vi "UHR-Fleezers Control (host) - 10.5.vi"() -> ()   [LabVIEW 2010]
uses:
  <vilib>/Utility/miscctls.llb/LVPoint32TypeDef.ctl
  <vilib>/Utility/miscctls.llb/LVMinMaxIncTypeDef.ctl
  openfpgaref.8.6.ctl
  <vilib>/userDefined/High Color/nirio_resource_hc.ctl
  <vilib>/Platform/TimedLoop/XDataNode/XDataNode.xnode
  <vilib>/Platform/TimedLoop/XDataNode/timing_clust.ctl
  <vilib>/Platform/TimedLoop/XDataNode/nitl_modes.ctl
  <vilib>/Platform/TimedLoop/XDataNode/wakeup.ctl
  <vilib>/rvi/interface/nirviOpenFPGA/nirviOpenFPGA.xnode
  FPGA Bitfiles/UHR-FleezersInst_FPGATarget_UHR-FleezersCont_0F5B06C4.lvbitx
  UHR-Fleezers Control (fpga) - 10.3.vi
  <vilib>/rvi/ClientSDK/nirviWhatTheDeviceIsDoing.ctl
  <vilib>/rvi/interface/nirviMethod/nirviMethod.xnode
  <vilib>/rvi/interface/nirviReadWriteControl/nirviReadWriteControl.xnode
  <vilib>/rvi/interface/common/niFpgaNodeNameForErrorReporting.ctl
  <vilib>/rvi/errors/niLvFpgaWhatHappensToTopLevelVI.ctl
  <vilib>/express/express analysis/Spectral/XNode/ExpressSpectralMeasurementsBlockNode.xnode
  <vilib>/rvi/interface/nirviCloseFPGA/nirviCloseFPGA.xnode
  <vilib>/Instr/_visa.llb/VISA Configure Serial Port (Instr).vi
  <vilib>/FPGAPlugInAG/PCIe-7852R/niLvFpga_Open_PCIe-7852R.vi
  <vilib>/FPGAPlugInAG/PCIe-7852R/niLvFpga_Reset_PCIe-7852R.vi
  <vilib>/Utility/error.llb/Error Cluster From Error Code.vi
  <vilib>/rvi/errors/niLvFpgaAdjustHostInterfaceError.vi
  <vilib>/express/express analysis/Spectral/Block/exnSpectralBlock spectral measurements PSD poly.vi
  <vilib>/express/express analysis/Spectral/Block/exnSpectralBlock spectral measurements PSD WFM.vi
  <vilib>/Waveform/WDTOps.llb/WDT Append Waveforms DBL.vi
  <vilib>/FPGAPlugInAG/PCIe-7852R/niLvFpga_Abort_PCIe-7852R.vi
  <vilib>/FPGAPlugInAG/PCIe-7852R/niLvFpga_Close_PCIe-7852R.vi
  <vilib>/Analysis/NI_AALBase.lvlib
  <vilib>/Platform/TimedLoop/XDataNode/XDNodeRunTimeDep.lvlib
  <vilib>/vision/NI_Vision_Development_Module.lvlib
  NiFpgaLv.dll
  <vilib>/Utility/inputDevices.llb/mouseAcquire.vi
  User32.dll
  <vilib>/Utility/inputDevices.llb/closeMouse.vi
panel:
  out "Array":cluster{i32, i32, i32, i32}[](array[cluster])
  in  "radius":i32
  in  "clear markers":bool
  in  "trap\nmarkers?":bool
  out "x-y":u32=299
  in  "Sample Channel Flow":bool
  in  "Pump 3 contents":string="Left: ADig beads" caption="contents"
  in  "Pump 1 contents":string="Right: DNA beads" caption="contents"
  in  "Scripts":T1(tab)
  in  "Take Stepping Data":bool
  in  "Cap 1 Samp Flow ON":bool=TRUE
  in  "Cap 2 Samp Flow ON":bool=TRUE
  in  "Got DNA bead":bool
  in  "Got ADig bead":bool
  in  "Cap 2 Flow ON":bool=TRUE
  in  "Cap 1 Flow ON":bool=TRUE
  in  "Cap 2 T ON":bool=TRUE
  in  "Move Cap. 2 (ADig Left)":bool
  in  "Move Cap. 1 (DNA Right)":bool
  in  "Cal/Data Acq. Spot":bool
  in  "Dump Beads":bool
  in  "Lower Ch. Cap.":bool
  in  "Cap 1 T ON":bool=TRUE
  in  "Offset 2 Set":dbl=2.0
  in  "Offset 1 Set":dbl
  in  "Cal @ (MHz)":dbl=15.0
  in  "W/ Offset 1":bool=TRUE
  in  "Offset 1 Start (MHz)":dbl=13.0
  in  "W/ Offset 2":bool=TRUE
  in  "Offset 2 Start (MHz)":dbl=16.0
  in  "Move to Delta 2 (MHz)":dbl=13.0
  in  "Attempt Limit":dbl=30.0 caption="Limit"
  out "Attempts":dbl=1.0
  in  "Wait Before Save (s)":u32=1
  in  "Fish for Tether":bool
  in  "Closest Delta (MHz)":dbl=9.5 step=0.25
  in  "Stop F (pN)":dbl=3.0
  in  "Then...":string(combo)="5"
  in  "Move to Delta 1 (MHz)":dbl=13.0
  in  "Tether Alarm?":bool=TRUE
  out "Tether":bool
  in  "TA Cancel Save?":bool=TRUE
  in  "TA Green Off?":bool=TRUE
  in  "Raster Set Upon Tether":u32=1
  in  "Save at end (5, 6)":bool
  in  "N Steps":dbl=20.0
  in  "Step Size (nm)":dbl=0.34
  in  "Save ave factor":dbl=1.0
  in  "Dip Trap Delta 1 (MHz)":dbl=15.0
  in  "Move Trap Before?":bool
  in  "Save Data After?":bool
  in  "Green ON After?":bool
  in  "Dip Trap Delta 2 (MHz)":dbl=15.0
  in  "Move Trap After?":bool
  in  "Duration (s)":dbl=1.0
  in  "Dip for Protein":bool
  in  "APD to Watch":bool
  out "Duration (s)":dbl
  in  "Action":string(combo)="Yank"
  in  "Fl. Triggered...":bool
  in  "Fl. Delta Thresh. (kHz)":dbl=0.6
  out "Waiting":bool
  out "Fl. High":bool
  in  "N pts to average":u16=6
  in  "Yank Delay (s)":dbl=3.5
  in  "Yank to Delta Array (MHz)":dbl[](array[numeric])=[16.3, 15.85, 14.85]
  in  "N Array El":u8=3 min=1 step=1
  in  "Random Choice":bool=TRUE
  in  "Force Yank":bool
  in  "Force Reset":bool
  in  "Y change (mm)":dbl
  in  "Profile":bool
  out "Sigma/Mean 2":dbl=nan caption="Sigma/Mean" format="%#_2g"
  out "Rate sigma (Hz) 2":dbl caption="Sigma (Hz)" format="%0.2f"
  out "APD 2 Rate (Hz)":dbl format="%#_3p"
  out "Primary Video Display":T2(plugin-control)
  out "Waveform Graph":dbl[](graph) caption="APD Line Scan"
  in  "Inject Pump 3":bool
  in  "Inject Pump 1":bool
  out "Messages":string="1:35 PM\tUHR-Fleezers ready.\r"
  in  "APD Ave N":dbl=10.0
  out "Int. Time (s)":dbl=3.0
  in  "Stop All":bool=TRUE
  out "Sigma/Mean":dbl=nan format="%#_2g"
  out "Rate sigma (Hz)":dbl caption="Sigma (Hz)" format="%0.2f"
  in  "Tab Control 6":T3(tab)
  in  "APD 2 Offset":dbl
  in  "APD 1 Offset":dbl
  out "RMS (Ang)":dbl=546.1615219992773 format="%_2g"
  in  "Bead Sep. Int. Time (s)":dbl=5.0 caption="Int. Time (s)"
  in  "Below (kHz)":dbl=0.5
  in  "Above (kHz)":dbl=2.0
  in  "Adjust Scale\nto Mean":bool
  in  "Rescale on Mean":bool
  in  "Offset (nm)":dbl
  out "Mean":dbl=25212.28425909567 caption="Mean (pN)" format="%#_3g"
  out "Force":waveform(dbl)[](graph)=[{"t0"=timestamp(535.5000000000101 s since 1904-01-01), "dt"=0.15, "Y"=[-25044.15793114605, -24955.246811984947], "attributes"=variant("NI_ChannelName"=variant(string "T1 X"))}, {"t0"=timestamp(535.5000000000101 s since 1904-01-01), "dt"=0.15, "Y"=[25464.576033689078, 25385.15625956261], "attributes"=variant("NI_ChannelName"=variant(string "T2 X"))}]
  out "APD Chart":waveform(dbl)[](graph)=[{"t0"=timestamp(535.5000000000101 s since 1904-01-01), "dt"=0.15, "Y"=[0.0, 0.0], "attributes"=variant("NI_ChannelName"=variant(string "APD 1"))}, {"t0"=timestamp(535.5000000000101 s since 1904-01-01), "dt"=0.15, "Y"=[0.0, 0.0], "attributes"=variant("NI_ChannelName"=variant(string "APD 2"))}]
  in  "Calibration":u16(ring)=2 items=["None", "Position", "Force"]
  out "T1 X":dbl=-24999.702371565498 caption="T1 X (pN)" format="%0.2f"
  out "T2 X":dbl=-25424.86614662584 caption="T2 X (pN)" format="%0.2f"
  out "Bead Separation":waveform(dbl)(graph)={"t0"=timestamp(535.5000000000101 s since 1904-01-01), "dt"=0.15, "Y"=[-15812.773305948416, -15807.156067093601], "attributes"=variant("NI_ChannelName"=variant(string "T1 X"))}
  in  "Amplitude (nm)":dbl=3.0
  out "Bead Mean (nm)":dbl=-15802.026676207124 caption="Mean (nm)" format="%0.2f"
  out "Difference":dbl=-425.16377506034405 caption="Difference (pN)" format="%.2g"
  in  "Take Detection Laser\nImage":bool
  out "APD 2":T2(plugin-control) caption="APD 2 (Cy5)"
  in  "Flip Green Filter":bool
  in  "Set X Only":bool
  in  "Set Y Only":bool
  out "APD 1":T2(plugin-control) caption="APD 1 (Cy3)"
  out "Detection Laser Y":T2(plugin-control)
  out "Pointer Y (V)":dbl format="%_3g"
  out "Pointer X (V)":dbl format="%_3g"
  in  "Set Confocal Spot (X-Y)":bool
  out "Detection Laser X":T2(plugin-control)
  out "Saved APD":dbl[][](graph) caption="Most Recent Time Trace"
  out "Trap Delta Graph":dbl[](graph)=[nan, nan, nan, nan, nan, nan, nan, nan, nan, nan, nan, nan, nan, nan, nan, nan, nan, nan, 5506.783124198511, -4646.991794395508, -35694.43968207309, -35619.5772041491, -35821.91480216695, -35730.943178839574, -35504.898467565145, -35354.8804233656, -35472.76573700478, -35401.34607848484, -35388.089521316375, -35339.12134773182, -35459.199275201856, -35729.41895938288, -35689.39427388793, -35652.754800380106, -35436.772050958185, -35739.738597278134, -35608.414119129695, -35743.24613971659, -35784.38382085103, -35716.59751512454, -35815.93923548916, -35775.95454279274, -35779.23619593948, -35484.77470564126, -35327.609264795086, -34995.24495804135, -35416.78159850549, -35725.53692538933, -35748.079800634034, -35880.92836793301, -35749.78262354857, -35978.67320672986, -35869.0014248518, -35789.42492120524, -35757.0094743559, -35665.61831994797, -35820.03745704799, -35862.82963519241, -35727.03914987952, -36026.712537387895, -36436.318288334776, -36401.456127681304, -36041.63767466281, -35954.18317002438, -35724.92232964981, -35868.8686397555, -35883.24492617235, -35803.0601673823, -35708.26805123931, -35799.06205723081, -35611.081301829865, -36272.35136131683, -36959.213279604824, -37036.11598280091, -36454.75633320364, -36363.13636613138, -36610.47217327304, -36856.865968068785, -36862.8035318567, -36611.41698123743, -36883.34140564069, -36809.41246397518, -36649.82010616029, -36608.216645825, -36263.2958780059, -36226.19432594783, -36303.70260886224, -37102.14814808201, -36292.439046917294, -35598.9894174926, -35830.98169581103, -36058.83611516422, -36225.468131644884, -36127.762280651485, -36082.00007470389, -36044.73871590373, -36150.75015432433, -36388.90061704641, -36444.12746082022, -36483.61738865511, -36918.38420800894, -39301.58608376002, -37410.88074835588, -36308.2937993105, -36276.00757609446, -36242.688728589026, -36279.07673698377, -36239.69924062693, -36115.100330006506, -36132.43861434632, -36216.16581615104, -36106.03516807985, -36124.044387950256, -36128.888004293534, -36577.72597656725, -36607.9878442394, -36823.0312420711, -36927.94596675817, -36723.10019041813, -36735.17581417585, -36642.46055551911, -36591.93053329535, -36830.67865023586, -36687.573975087755, -36279.003642519325, -36204.55551062233, -36162.4900595779, -36112.882352923174, -35845.751830077366, -35886.977427864345, -36246.00229479818, -36527.2689457434, -36126.69225184011, -36246.12051545762, -36512.13150467549, -36637.56546718613, nan, nan, nan, nan, nan, nan, nan, nan, nan, nan, nan, nan, nan, nan, nan, nan, 6167.109856754105, 5333.346252800504, 4786.115038807911, 5468.273126568616, 5516.36557661368, 5542.373796865417, 6078.611773943747, 5891.714844203729, 5618.914400659502, 5585.039741950386, 5230.524430755409, 5019.637598752583, 5565.129008078686, 5594.435284303661, 5479.090270436311, 5461.786221622111, 5521.225380142801, 5501.030997575479, 5853.9403315680975, 6277.41888789479, 6347.663416123396, 6518.521533988649, 6402.083920679695, 5586.7838515403855, 5555.057847331831, 6088.912612467204, 6103.1354775714135, 5433.827126832315, 5184.193155816407, 5200.778003036132, 5198.84830591151, 5216.670816959944, 4951.851075846338, 4809.302118575521, 5108.190699540166, 5368.621823883703, 5512.198704715542, 5093.721604642531, 4559.550615448883, 5100.95481291585, 5056.548567619509, 4941.672631440189, 5294.489502868484, 5186.6750265414885, 5292.553597092265, 5409.090662323695, 5306.546960408101, 5093.291555042684, 5132.176339256024, 5136.5655798997905, 5074.835794252038, 5191.191273408171, 6355.507410750361, 4835.374250389592, 4857.78217273175, 4720.100040370948, 4959.276993173975, 5063.446039367191, 4977.321913173073, 5109.219099074602, 5152.93064060052, 5547.020563293438, 5641.477304542917, 5522.296307770564, 5375.801023327964, 5397.33578156725, 5739.127097393721, 5473.835813570375, 5092.189342098223, 5078.737073516502, 5108.415259040703, 4688.592359177841, 4194.126176561986, 4543.527821563446, 4318.231193368585, 4242.50202161097, 3927.9613565170293, 3892.7267486210185, 4066.225930797533, 4065.91368279951, 4284.926895395256, 4413.920454823281, 4682.053196625115, 4645.313376230479, 4787.871154537963, 4620.104593196258, 4689.874618170274, 4574.540529970007, 4550.143507058878, 4282.883067791481, 4262.784558608793, 4658.908267837964, 4624.420048893822, 4545.280989238992, 4534.685165027797, 4509.55138972502, 4836.356510905302, 4816.034613159383, 4735.337933910836, 4557.19809251558, 4379.409787660465, 4815.099334183324, 4958.8354348926805, 5277.922068526226, 5478.752691463218, 5386.796035256921, 5304.423898437439, 5140.107866682738, 4629.225225550923, 4495.885935607061, 4585.106123752586, 4020.716761082964, 3869.455949078052, 3775.6939108328515, 4283.506628339179, 4255.9895575880655, 4207.326476232527, 4481.910554085669, 4290.552944524519, 4300.538092951319, 4262.93523584069, 4124.084931480189, 4145.961534257469, 4469.723898944911, 4257.080867276527, 4584.2495480337675, 4878.593776781403, 4862.389773302828, 4424.025610809404, 5015.237366030138, 5368.934630101561, 5268.2358864831185, 5270.762456451324, 5071.971107422025, 4788.286125615632, 5068.804170150252, 5635.453206195743, 5300.26545412367, 5053.7452073194, 4411.6408011639, 4729.437948013554, 4616.721712242477, 4217.560168632146, 1853.2956126724166, 2731.4495324884047, 1965.8304299075971, 1681.1816010433686, 3900.1059432742477, 4508.806743955953, 4540.685808228605, 4394.341315410638, 4332.994739636473, 4619.785713311023, 4682.894381776627, 4590.441265195375, 4592.289661643896, 4517.628053144901, 4521.989999556128, 4153.759374101326, 4217.3744770279445, 4254.7495631356, 4517.795825609486, 4792.4222714998905, 4848.140062460021, 4872.213524688195, 4296.270859130964, 4287.140354177507, 4271.232522639795, 4086.2294053148507, 4066.054335077002, 3369.498673954018, 3399.8636469264748, 4266.888719325172, 4182.548037886663, 3611.537869539432, 4010.20848817387, 4597.454566559376, 4355.452743049478, 4694.424339866659, 4872.450870939836, 4835.863789324721, 4944.1445064812, 5029.996116973678, 4874.364145354353, 4115.32227349357, 3795.149770730146, 3748.0286024254456, 3844.4840368036384, 3783.022889138141, 3404.701132355549, 3376.389749611073, 3466.8981377561868, 3586.1944526531443, 3696.545814003315, 3611.3565660750755, 3679.737914768004, 3666.7967692377424, 3676.711590811392, 3657.090966472111, 4046.639438605751, 4243.416804539156, 4330.018049953724, 4005.8202012123074, 3886.8678397881595, 3936.7748002889566, 4414.532217689804, 4460.044591326805, 4667.592778086604, 4554.681804379012, 4525.9256994475, 4535.175121351291, 4640.441589664973, 4463.295761819958, 4299.017081874554, 4344.679534951516, 4159.076084998815, 4258.264845617887, 4342.03723123527, 4293.802608954749, 4257.300224741368, 4109.126840762474, 4284.031531368601, 4207.8796632743615, 4100.048772335067, 4087.96379355331, 4260.744316169628, 4256.3750247303105, 3965.8701192156004, 3542.1177219529345, 3245.9072470112296, 3260.3512171382317, 2722.9535738104023, 2617.7212182873336, 2495.4361735372368, 2480.0800319289992, 2166.2326383851178, 1837.2762906802964, 1561.7085528177995, 2009.358375284457, 2421.4478925286967, 3333.165825583201, 2478.103570909574, 2670.9941767873534, 2912.4602155767498, 3272.8857489395596, 3283.649132292325, 3348.3640076944575, 3237.5396827965596, 2990.6844306564017, 2961.4708811208548, 3051.669620746834, 2803.3078944807203, 2639.8891909174854, 2697.3504137075943, 2528.713908432488, 2574.636537743907, 2694.1698351749073, 2309.540812026258, 1697.3556335092435, 1944.4873971808265, 1886.9800885020231, 1780.5991255762056, 1447.55923768894, 1184.8594220131345, 1270.5842650151462, 1701.1096547279885, 1682.135100016123, 1465.440496745956, 1458.9290230144252, 1495.4322015184443, 1565.122029892751, 1326.2808670992672, 2430.0063374171295, 1366.999249788816, 1511.7599002618226, 1537.5122448183974, 1528.379436629737, 1576.0772089301026, 1661.463700236185, 1633.6669499352138, 1550.5369732750987, 1618.08719272913, 1735.053686743573, 1528.4256208017614, 1359.678346291199, 1448.879271423386, 1698.6632704650692, 1744.61641698936, 1737.8936943446897, 1647.717667490957, 1713.8264302250027, 1634.9713900046336, 1602.5970094116783, 1346.5591554460843, 1236.9326521952025, 1248.729790403464, 1239.3985080938874, 860.3757220196276, 309.03249515453354, 872.3440498684358, 1070.4760944124719, 1025.611590261964, 762.536767328711, 519.0841121808917, 528.9937890777801, 628.9594749419193, 752.1756994154857, 346.70657858092454, 603.7321641918679, 872.6109227435372, 718.0242704203702, 480.7930988375738, 623.1033508402033, 730.0590904870769, 863.1542840743932, 1057.2107828814624, 1282.580174010378, 1150.575729720411, 958.504006769319, 718.2215734648926, 336.9203146637883, 499.64211424942187, 489.86888967592677, 515.8774775462225, 401.9460443397984, 428.7305987011496, 559.0300917017885, 698.674723764605, 863.9018844876991, 1621.2053660150123, 842.1787038501789, 865.7734767645452, 747.962438460745, 937.7230403821741, 862.8234610329819, 880.4157930621295, 686.8554584070225, 698.575513254953, 582.4487325239024, 879.2979023331573, 1084.1922318673605, 800.0059949128045, 872.6097495401191, 1575.7345694812684, -13.817523221398005, 186.55566427808662, 141.7235428805143, 33.77184446551837, 69.20933341039927, -1.0905661626020446, -33.63782661705045, -7.14325079334958, 93.77236987595097, 25.515056188742165, 37.78173931318452, 256.93076609475247, 534.7722772616544, 747.3287373992207, 677.6056943976873, 651.2208013388299, 729.420141819006, 824.8649777809915, 929.2410418248328, 928.5734546254243, 917.3695968623797, 864.3437715625332, 1276.7402930616954, 1531.80179383418, 1615.8453486703365, 1696.5065934156737, 1479.2476703459397, 1362.4142350116745, 1460.847270054117, 1374.8810863509425, 1381.447829146564, 1265.5623497677589, 1158.3770254538977, 1165.2760177916934, 1301.4281341239985, 1164.6825921675918, 654.6588563997066, 626.5015050760849, 506.6957864504802, 697.5467290992237, 792.5745738661499, 839.1173683659872, 653.3795353904134, 512.1537277876778, 494.6333207292337, 510.5975695020461, 374.8426834060956, 438.63421711552655, 291.18890517803084, 872.5884805703972, 1076.141667530479, 1100.179772342759] caption="Most Recent Time Trace"
  out "Save APD Deriv":dbl[][](graph) caption="Most Recent Time Trace"
  out "Delta Fl. 1":dbl
  out "Delta Fl. 2":dbl
  out "All Signals":waveform(dbl)[](graph)=[{"t0"=timestamp(535.5000000000101 s since 1904-01-01), "dt"=0.15, "Y"=[0.0, 0.0], "attributes"=variant("NI_ChannelName"=variant(string "APD 1"))}, {"t0"=timestamp(535.5000000000101 s since 1904-01-01), "dt"=0.15, "Y"=[0.0, 0.0], "attributes"=variant("NI_ChannelName"=variant(string "APD 2"))}, {"t0"=timestamp(535.5000000000101 s since 1904-01-01), "dt"=0.15, "Y"=[-13.234937024494576, -13.036495504338259], "attributes"=variant("NI_ChannelName"=variant(string "T1 Y"))}, {"t0"=timestamp(535.5000000000101 s since 1904-01-01), "dt"=0.15, "Y"=[-148.5348487150217, -148.00768403325296], "attributes"=variant("NI_ChannelName"=variant(string "T1 X"))}, {"t0"=timestamp(535.5000000000101 s since 1904-01-01), "dt"=0.15, "Y"=[-0.014816858424634217, -0.014869899594103498], "attributes"=variant("NI_ChannelName"=variant(string "T1 Sum"))}, {"t0"=timestamp(535.5000000000101 s since 1904-01-01), "dt"=0.15, "Y"=[-42.33660401340703, -41.80386077646538], "attributes"=variant("NI_ChannelName"=variant(string "T2 Y"))}, {"t0"=timestamp(535.5000000000101 s since 1904-01-01), "dt"=0.15, "Y"=[-148.2704140029845, -147.8081260018218], "attributes"=variant("NI_ChannelName"=variant(string "T2 X"))}, {"t0"=timestamp(535.5000000000101 s since 1904-01-01), "dt"=0.15, "Y"=[-0.014843317972349905, -0.014889980773338704], "attributes"=variant("NI_ChannelName"=variant(string "T2 Sum"))}, {"t0"=timestamp(535.5000000000101 s since 1904-01-01), "dt"=0.15, "Y"=[-inf, -inf], "attributes"=variant("NI_ChannelName"=variant(string "T1 FB X"))}, {"t0"=timestamp(535.5000000000101 s since 1904-01-01), "dt"=0.15, "Y"=[-0.00023483993041779493, -0.00022965178380687546], "attributes"=variant("NI_ChannelName"=variant(string "T1 FB Sum"))}, {"t0"=timestamp(535.5000000000101 s since 1904-01-01), "dt"=0.15, "Y"=[-inf, -inf], "attributes"=variant("NI_ChannelName"=variant(string "T2 FB X"))}, {"t0"=timestamp(535.5000000000101 s since 1904-01-01), "dt"=0.15, "Y"=[-0.00016696676534317856, -0.00016208380382701907], "attributes"=variant("NI_ChannelName"=variant(string "T2 FB Sum"))}, {"t0"=timestamp(535.5000000000101 s since 1904-01-01), "dt"=0.15, "Y"=[-0.0197486346190042, -0.015821571005484064], "attributes"=variant("NI_ChannelName"=variant(string "PSD Y"))}, {"t0"=timestamp(535.5000000000101 s since 1904-01-01), "dt"=0.15, "Y"=[-0.30516096686887967, -0.3022235108217065], "attributes"=variant("NI_ChannelName"=variant(string "PSD X"))}, {"t0"=timestamp(535.5000000000101 s since 1904-01-01), "dt"=0.15, "Y"=[-0.007494613483077324, -0.007518753624072838], "attributes"=variant("NI_ChannelName"=variant(string "PSD Y Sum"))}]
  in  "Signals to Plot":i32(listbox)
  out "Trap Disp. Freq. (Hz)":dbl=6.666666666666667 caption="Freq. (Hz)" format="%#_6p"
  out "Display Period (s)":dbl=0.15 caption="Period (s)" format="%#_6p"
  in  "Trap Disp. Downsample":dbl=10000.0 caption="Downsample" max=20000.0
  in  "APD Disp. Scale":dbl=0.1 caption="Scale (Divide,\nfor above plot only)"
  in  "APD Disp. Downsample":dbl=15.0 caption="Integrate" min=1.0 max=30.0 step=1.0
  out "APD Display Freq. (Hz)":dbl=6.666666666666667 caption="Freq. (Hz)"
  out "APD Display Period (s)":dbl=0.15 caption="Period (s)"
  out "FFT 1":cluster{"f0":dbl, "df":dbl, "magnitude":dbl[]}[](graph)=[{"f0"=0.0, "df"=3.3333333333333335, "magnitude"=array[10000 elements]}, {"f0"=0.0, "df"=3.3333333333333335, "magnitude"=array[10000 elements]}]
  out "FFT 2":cluster{"f0":dbl, "df":dbl, "magnitude":dbl[]}[](graph)=[{"f0"=0.0, "df"=3.3333333333333335, "magnitude"=array[10000 elements]}, {"f0"=0.0, "df"=3.3333333333333335, "magnitude"=array[10000 elements]}]
  in  "FFT 1 Choice 1":u16(ring) items=["T1 Y", "T1 X", "T1 Sum", "T2 Y", "T2 X", "T2 Sum", "T1 FB Y", "T1 FB X", "T1 FB Sum", "T2 FB Y", "T2 FB X", "T2 FB Sum", "PSD X", "PSD Y Sum", "none"]
  in  "FFT 2 Choice 1":u16(ring)=3 items=["T1 Y", "T1 X", "T1 Sum", "T2 Y", "T2 X", "T2 Sum", "T1 FB Y", "T1 FB X", "T1 FB Sum", "T2 FB Y", "T2 FB X", "T2 FB Sum", "PSD X", "PSD Y Sum", "none"]
  in  "FFT 1 Choice 2":u16(ring)=1 items=["T1 Y", "T1 X", "T1 Sum", "T2 Y", "T2 X", "T2 Sum", "T1 FB Y", "T1 FB X", "T1 FB Sum", "T2 FB Y", "T2 FB X", "T2 FB Sum", "PSD X", "PSD Y Sum", "none"]
  in  "FFT 2 Choice 2":u16(ring)=4 items=["T1 Y", "T1 X", "T1 Sum", "T2 Y", "T2 X", "T2 Sum", "T1 FB Y", "T1 FB X", "T1 FB Sum", "T2 FB Y", "T2 FB X", "T2 FB Sum", "PSD X", "PSD Y Sum", "none"]
  in  "Compute FFT":bool=TRUE
  in  "Reset FFT":bool
  in  "# Spectra to Ave.":dbl=25.0
  out "Ave. Time (s)":dbl=7.5
  out "1 Channel":waveform(dbl)(graph)={"t0"=timestamp(0 s since 1904-01-01), "dt"=1.4999999999999999e-05, "Y"=array[20000 elements], "attributes"=variant("NI_ChannelName"=variant(string "T1 Y"))}
  out "Slow mean":dbl=0.04741485510254009 format="%0.2f"
  in  "Slow mean N ave.":dbl=1.0 min=1.0 step=1.0
  out "Mean Intensity":dbl=0.04741485510254009
  out "Sigma":dbl=0.006116447585273888
  out "Sigma/Mean":dbl=0.12899855060289364
  in  "Subtract mean":bool
  in  "High Res. Display":u16(ring) items=["T1 Y", "T1 X", "T1 Sum", "T2 Y", "T2 X", "T2 Sum", "T1 FB Y", "T1 FB X", "T1 FB Sum", "T2 FB Y", "T2 FB X", "T2 FB Sum", "PSD X", "PSD Y Sum"]
  out "APD 1 Rate (Hz)":dbl format="%#_3p"
  in  "Tab Control":T4(tab)=enum."Trap Control (RF)"
  out "Stage Moving":bool
  in  "Read Cal":bool
  in  "Confocal Linescan":bool
  in  "Speed (nm/s)":dbl=100.0
  in  "Furthest Withdraw (MHz)":dbl=15.0
  in  "Confocal Image":bool
  in  "Round T1 X":bool caption="Round"
  in  "T1 offset_x (mV)":dbl=-45.0347243000155 format="%#_2g"
  in  "T1 kappa_x (pN/nm)":dbl=0.2471971927099238 min=0.0 step=0.001 format="%#_2g"
  out "Time (s)":dbl=62.099999999999994
  out "Total Time (s)":dbl=60.0
  in  "Start Saving":bool
  in  "Cal sets to save":u32=50 min=1 step=1
  in  "Comment (data description)":string="testing confocal setup"
  out "Calibrating Trap...":bool
  in  "Trap 2 (ON/OFF)":bool=TRUE
  in  "Trap 1 (ON/OFF)":bool=TRUE
  in  "Save Calibration":bool
  in  "N sets to save":u32=200 caption="N Sets"
  in  "Save N Sets":bool
  out "Save file name":path=path "C:/Data/110512/110512_002.dat"
  in  "Save ave N":dbl=500.0 caption="Averaging Factor"
  out "Saving...":bool
  in  "Stop Saving":bool
  out "Progress":u16(slide) scale=0.0..100.0
  out "Manipulating Trap":bool
  out "Buffer Status":dbl(slide)=1.1666666666666666e-05 scale=0.0..1.0
  out "Overflow (data lost)":bool
  in  "Reset":bool
  out "Data Rate (Hz)":dbl=66666.66666666667 caption="Trap Data Rate (Hz)" format="%#_3p"
  out "Data Period (s)":dbl=1.4999999999999999e-05 caption="Trap Data Period (s)" format="%#_6p"
  out "Save Data Rate (Hz)":dbl=133.33333333333334 caption="Rate (Hz)" format="%#_6p"
  out "Save Data Period (s)":dbl=0.0075 caption="Period (s)" format="%#_6p"
  in  "T1 alpha_x (nm/V)":dbl=682.2856484824291 step=10.0 format="%#_3g"
  in  "T2 alpha_x (nm/V)":dbl=790.1873608955543 step=10.0 format="%#_3g"
  in  "T2 kappa_x (pN/nm)":dbl=0.2174132196053945 min=0.0 step=0.001 format="%#_2g"
  in  "T2 offset_x (mV)":dbl=-45.767376265464655 format="%#_2g"
  in  "BD 1 Frequency 2 (MHz)":dbl=90.0 caption="T2 X (MHz)" min=60.0 max=90.0 step=1.0 format="%#_6p"
  in  "Green Laser ON/Interlacing":bool
  in  "Round T2 X":bool caption="Round"
  in  "AO1":dbl(slide)=6.408063513378007 caption="Confocal Y (V)" min=0.0 max=10.0 step=0.01 scale=0.0..10.0 scale format="%_1f"
  in  "AO2":dbl(slide)=2.4332770775475328 caption="Confocal X (V)" min=0.0 max=10.0 step=0.01 scale=0.0..10.0 scale format="%_1f"
  in  "Trap Raster Scan":bool
  out "Raster Scanning...":bool
  in  "Trap Delta (MHz)":dbl=30.0
  in  "Trap Intensity\nSetpoints (V)":cluster{"Set 1":dbl, "Set 2":dbl}={"Set 1"=2.2, "Set 2"=2.2}
  in  "Index":dbl=1.0 caption="Save File Index" min=1.0 step=1.0
  in  "BD 1 Frequency 1 (MHz)":dbl=60.0 caption="T1 X (MHz)" min=60.0 max=90.0 step=1.0 format="%#_6p"
  in  "reset motor comm. link":bool
  out "Waveform Chart":T5(graph)={"Current Position[0]"=0.0, "Current Position[1]"=5.75288266, "Current Position[2]"=6.13417492, "Current Position[3]"=0.0, "Current Position[4]"=0.0, "Current Position[5]"=0.0, "Current Position[6]"=0.0, "Current Position[7]"=0.0, "Current Position[8]"=0.0}
  out "Current Position":dbl[](array[numeric])=[0.0, 5.75288266, 6.13417492] format="%7_7g"
  in  "invert y?":bool
  in  "invert x?":bool=TRUE
  in  "mouse sensitivity":dbl(slide)=4.94949494949495 scale=0.0..10.0
  in  "Use mouse to move stage\n(press any key to quit)":bool
  in  "Position Label 5":string="upper flow spot (UvrD)" caption="5"
  in  "Move to Position":bool
  in  "Position":dbl=1.0 min=1.0 max=10.0 step=1.0
  in  "Set Position":bool
  in  "Saved Stage Positions":dbl[][](array[numeric])=[[1.0, 7.2685, 5.873467, 6.11521279], [2.0, 6.0401, 5.2271309, 6.10430308], [3.0, 7.0617, 5.85593148, 5.86877634], [4.0, 8.7609, 5.85593148, 5.86880685], [5.0, 6.0, 6.0, 6.0], [6.0, 0.0, 0.0, 0.0], [7.0, 0.0, 0.0, 0.0], [8.0, 0.0, 0.0, 0.0], [9.0, 0.0, 0.0, 0.0], [10.0, 0.0, 0.0, 0.0]]
  in  "Move to Position 5":bool
  in  "z nudge increment (um)":dbl=3.0
  in  "+z":bool
  in  "Position 1 Label":string="Right capillary (DNA beads)" caption="1"
  in  "Set Position 1":bool
  in  "Set Position 2":bool
  in  "Set Position 3":bool
  in  "Set Position 4":bool
  in  "Move to Position 3":bool
  in  "Move to Position 4":bool
  in  "Move to Position 2":bool
  in  "Move to Position 1":bool
  in  "Position 2 Label":string="Left capillary (ADig beads)" caption="2"
  in  "Position 3 Label":string="lower flow spot (ATP)" caption="3"
  in  "Position 4 Label":string="Dump beads" caption="4"
  in  "-z":bool
  in  "Set Position 5":bool
  in  "lateral step size (mm)":dbl=0.1
  out "Pump 3 cont disp":string="Left: ADig beads"
  out "Pump 1 cont disp":string="Right: DNA beads "
  in  "Ch 1 Inject Rate (ul/h)":dbl=50.0
  in  "Pump write delay (ms)":dbl=300.0
  in  "All Pump Parameters":T6={"Pump 1"={"Diameter (mm)"=4.61, "Units"=4.0, "Volume"=100.0, "Rate"=50.0}, "Pump 2"={"Diameter (mm)"=4.61, "Units"=3.0, "Volume"=0.0, "Rate"=0.0}, "Pump 3"={"Diameter (mm)"=4.61, "Units"=4.0, "Volume"=100.0, "Rate"=250.0}}
  in  "Ch 2 Inject Volume (uL)":dbl=100.0
  in  "Pump pause delay (ms)":u32
  in  "Ch 3 Inject Volume (uL)":dbl=100.0
  in  "Ch 3 Inject Rate (ul/h)":dbl=250.0
  in  "Flush Center Ch Volume (uL)":dbl=15.0
  in  "Flush Center Ch Rate (ul/m)":dbl=100.0
  in  "Inject Pump 2":bool caption="Inject Pump 2\n(Flush Center)"
  in  "Total Volume\nFlushed (uL)":dbl
  in  "Tab Control 2":T7(tab)=enum."Feedback on Trap Intensity"
  out "Total Counts (ticks)":u32=600
  in  "Trap ON/OFF X or Y Amp?":bool=TRUE
  in  "Oscillate Set 1":bool
  in  "Trap 1 ON":bool=TRUE
  in  "Number Interlace Sets":u8=3 min=1 max=3
  in  "DIO count 3 (ticks)":u32=200
  in  "DIO count 2 (ticks)":u32=200
  in  "DIO count 1 (ticks)":u32=200
  in  "BD 2 Amplitude 3 (%)":dbl min=0.0 max=50.0 step=1.0
  in  "BD 2 Amplitude 2 (%)":dbl min=0.0 max=50.0 step=1.0
  in  "BD 2 Amplitude 1 (%)":dbl min=0.0 max=50.0 step=1.0
  in  "BD 1 Amplitude 3 (%)":dbl min=0.0 max=50.0 step=1.0
  in  "BD 1 Amplitude 2 (%)":dbl=30.0 min=0.0 max=50.0 step=1.0
  in  "BD 1 Amplitude 1 (%)":dbl=35.0 min=0.0 max=50.0 step=1.0
  in  "BD 2 Frequency 3 (MHz)":dbl=26.0 min=0.0 max=40.0 step=1.0 format="%#_6p"
  in  "BD 1 Frequency 3 (MHz)":dbl=70.0 min=60.0 max=90.0 step=1.0 format="%#_6p"
  in  "BD 2 Frequency 2 (MHz)":dbl=26.0 min=0.0 max=40.0 step=1.0 format="%#_6p"
  in  "BD 2 Frequency 1 (MHz)":dbl=26.0 min=0.0 max=40.0 step=1.0 format="%#_6p"
  in  "Not-Interlacing Set":enum32{"Set 1", "Set 2", "Set 3"}(radio)
  in  "Interlace":bool=TRUE
  in  "Trap 2 ON":bool=TRUE
  in  "Trap 3 ON":bool
  in  "Scan axis 2":bool=TRUE
  in  "Osc. freq. (Hz)":dbl=0.25
  in  "Osc. amp. (MHz)":dbl=2.0 format="%1_3g"
  out "Coords":T8
  in  "Manipulation Scaling":cluster{"Horizontal":dbl, "Vertical":dbl}={"Horizontal"=0.075, "Vertical"=0.01}
  in  "Freq or Amp switch first":bool=TRUE
  in  "Swap F1 and F2":bool
  in  "Freq switch delay":u16
  in  "Amp switch delay":u16=5
  in  "MCL Step Increment (V_int)":dbl=3.0
  out "Time to Finish All (min)":dbl=6.02946 format="%#_2p"
  in  "Scan Speed (nm/s)":dbl=1.36
  in  "Scan Range (nm)":dbl=-245.99999999999966
  in  "Step Size (nm)":dbl=1.0
  in  "MCL/AOM Scale Tweak":dbl=1.0
  in  "MCL Step Position Ratio":dbl=0.5
  in  "Move MCL Also?":bool=TRUE
  out "Final sep (nm)":dbl=2619.0
  out "Initial sep (nm)":dbl=2865.0
  out "Save index":dbl=2.0
  out "Final delta (MHz)":dbl=28.0
  out "Initial delta (MHz)":dbl=30.0
  out "Final freq. (MHz)":dbl=62.0
  out "Initial freq. (MHz)":dbl=60.0
  in  "Saved AOD Raster Scan Parameter Sets":T9(array[cluster])=[{"Scan Range AOD (nm) 2"=500.0, "Step Size AOD (nm) 2"=1.0, "Scan Speed AOD (nm/s) 2"=100.0, "Number of scans (AOD) 2"=1, "Label"="offset curve"}, {"Scan Range AOD (nm) 2"=420.0, "Step Size AOD (nm) 2"=1.0, "Scan Speed AOD (nm/s) 2"=100.0, "Number of scans (AOD) 2"=1, "Label"="hp raster check"}, {"Scan Range AOD (nm) 2"=6.8, "Step Size AOD (nm) 2"=0.34, "Scan Speed AOD (nm/s) 2"=0.34, "Number of scans (AOD) 2"=1, "Label"="3.4 kbp - 1 bp steps"}]
  in  "Load parameters":bool
  out "Scan Range (MHz)":dbl=1.9999999999999973
  in  "Restart DMA? (AOD)":bool=TRUE caption="Restart DMA?"
  out "Incr. int (AOD)":i64=7759651845
  out "Time/Scan (s) (AOD)":dbl=180.8838 format="%#_2p"
  out "Data points/scans":dbl=24117840.0
  out "Data points/scan (f/b)":dbl=24117840.0
  in  "Save scans":bool=TRUE
  out "AOD Scan I":u64 caption="Scan I"
  in  "Continuous AOD Scanning":bool caption="Continuous Scanning"